vi "Dresden R2R Sputter 03.02.2018 IY24.vi"() -> ()   [LabVIEW 2009] (continued)
                                frame #1 {
                                n20568 = local read "Semi"() -> (w23364:bool)
                                n20569 = case shown="False" w23364 {
                                frame #0 {
                                n20570 = Wait (ms)(milliseconds to wait=u32 1000) -> ()  [unwired: 1 out]
                                n20571 = local write "Ch3_Sd3"(TRUE ("Ch1_Sd1 2")) -> ()
                                }
                                frame #1 {
                                }
                                }
                                }
                                }
                                }
                                frame #1 {
                                }
                                }
                              }
                              frame #4 {
                                n20572 = local read "Yes 3"() -> (w23367:bool)
                                n20573 = case shown="False" w23367 {
                                frame #0 {
                                # "CLOSE PC-BV"
                                n20574 = local read "Semi"() -> (w23368:bool)
                                n20575 = case shown="False" w23368 {
                                frame #0 {
                                n20576 = stacked-sequence {
                                frame #0 {
                                n20577 = local read "Semi"() -> (w23369:bool)
                                n20578 = case shown="False" w23369 {
                                frame #0 {
                                n20579 = stacked-sequence {
                                frame #0 {
                                n20580 = local read "Semi"() -> (w23370:bool)
                                n20581 = case shown="False" w23370 {
                                frame #0 {
                                n20582 = local write "Pc_bv3_auto_close"(TRUE ("Tp1_auto_start")) -> ()
                                }
                                frame #1 {
                                }
                                }
                                }
                                frame #1 {
                                n20583 = local read "Semi"() -> (w23372:bool)
                                n20584 = case shown="False" w23372 {
                                frame #0 {
                                n20585 = Wait (ms)(milliseconds to wait=u32 1000) -> ()  [unwired: 1 out]
                                }
                                frame #1 {
                                }
                                }
                                }
                                frame #2 {
                                n20586 = local read "Semi"() -> (w23374:bool)
                                n20587 = case shown="False" w23374 {
                                frame #0 {
                                n20588 = while {
                                i -> [w23380]
                                stop <- w23376 stop-if-true
                                n20589 = local read "Pc_bv_closed_ch3"() -> (w23378:bool)
                                n20590 = Greater?(x=w23380, y=120) -> (0:w23379:bool)
                                n20591 = local read "Semi"() -> (w23377:bool)
                                n20592 = Compound Arithmetic op=OR(w23377, w23378, w23379) -> (w23376:bool)
                                n20593 = Wait (ms)(milliseconds to wait=u32 500) -> ()  [unwired: 1 out]
                                }
                                }
                                frame #1 {
                                }
                                }
                                }
                                frame #3 {
                                n20594 = local read "Semi"() -> (w23382:bool)
                                n20595 = case shown="False" w23382 {
                                frame #0 {
                                n20596 = local read "Pc_bv_closed_ch3"() -> (w23383:bool)
                                n20597 = case shown="False" w23383 {
                                frame #0 {
                                n20598 = local write "Pc_bv3_auto_close"(TRUE ("Pc_bv1_auto_open")) -> ()
                                }
                                frame #1 {
                                }
                                }
                                }
                                frame #1 {
                                }
                                }
                                }
                                frame #4 {
                                n20599 = local read "Semi"() -> (w23385:bool)
                                n20600 = case shown="False" w23385 {
                                frame #0 {
                                n20601 = local read "Pc_bv_closed_ch3"() -> (w23386:bool)
                                n20602 = case shown="False" w23386 {
                                frame #0 {
                                n20603 = Wait (ms)(milliseconds to wait=u32 1000) -> ()  [unwired: 1 out]
                                }
                                frame #1 {
                                }
                                }
                                }
                                frame #1 {
                                }
                                }
                                }
                                frame #5 {
                                n20604 = local read "Semi"() -> (w23388:bool)
                                n20605 = case shown="False" w23388 {
                                frame #0 {
                                n20606 = while {
                                i -> [w23394]
                                stop <- w23390 stop-if-true
                                n20607 = local read "Pc_bv_closed_ch3"() -> (w23392:bool)
                                n20608 = Greater?(x=w23394, y=120) -> (0:w23393:bool)
                                n20609 = local read "Semi"() -> (w23391:bool)
                                n20610 = Compound Arithmetic op=OR(w23391, w23392, w23393) -> (w23390:bool)
                                n20611 = Wait (ms)(milliseconds to wait=u32 500) -> ()  [unwired: 1 out]
                                }
                                }
                                frame #1 {
                                }
                                }
                                }
                                frame #6 {
                                n20612 = local read "Semi"() -> (w23396:bool)
                                n20613 = case shown="False" w23396 {
                                frame #0 {
                                n20614 = local read "Pc_bv_closed_ch3"() -> (w23397:bool)
                                n20615 = case shown="False" w23397 {
                                frame #0 {
                                n20616 = local write "Error Message"("Shut Down process  cancelled\nbecause  PC-BV not opened.\nPlease check PC-BV3 connections." ("Error Message")) -> ()
                                n20617 = local write "Semi"(TRUE ("Semi")) -> ()
                                }
                                frame #1 {
                                }
                                }
                                }
                                frame #1 {
                                }
                                }
                                }
                                }
                                }
                                frame #1 {
                                }
                                }
                                }
                                frame #1 {
                                n20618 = local read "Semi"() -> (w23400:bool)
                                n20619 = case shown="False" w23400 {
                                frame #0 {
                                n20620 = local write "Ch3_Sd4"(TRUE ("Ch1_Sd2")) -> ()
                                n20621 = Wait (ms)(milliseconds to wait=u32 1000) -> ()  [unwired: 1 out]
                                }
                                frame #1 {
                                }
                                }
                                }
                                }
                                }
                                frame #1 {
                                }
                                }
                                }
                                frame #1 {
                                # "OPEN PC-BV"
                                n20622 = local read "Semi"() -> (w23403:bool)
                                n20623 = case shown="False" w23403 {
                                frame #0 {
                                n20624 = stacked-sequence {
                                frame #0 {
                                n20625 = local read "Semi"() -> (w23404:bool)
                                n20626 = case shown="False" w23404 {
                                frame #0 {
                                n20627 = stacked-sequence {
                                frame #0 {
                                n20628 = local read "Semi"() -> (w23405:bool)
                                n20629 = case shown="False" w23405 {
                                frame #0 {
                                n20630 = local write "Pc_bv3_auto_open"(TRUE ("Tp1_auto_start")) -> ()
                                }
                                frame #1 {
                                }
                                }
                                }
                                frame #1 {
                                n20631 = local read "Semi"() -> (w23407:bool)
                                n20632 = case shown="False" w23407 {
                                frame #0 {
                                n20633 = Wait (ms)(milliseconds to wait=u32 1000) -> ()  [unwired: 1 out]
                                }
                                frame #1 {
                                }
                                }
                                }
                                frame #2 {
                                n20634 = local read "Semi"() -> (w23409:bool)
                                n20635 = case shown="False" w23409 {
                                frame #0 {
                                n20636 = while {
                                i -> [w23415]
                                stop <- w23411 stop-if-true
                                n20637 = local read "Pc_bv_opened_ch3"() -> (w23413:bool)
                                n20638 = Greater?(x=w23415, y=120) -> (0:w23414:bool)
                                n20639 = local read "Semi"() -> (w23412:bool)
                                n20640 = Compound Arithmetic op=OR(w23412, w23413, w23414) -> (w23411:bool)
                                n20641 = Wait (ms)(milliseconds to wait=u32 500) -> ()  [unwired: 1 out]
                                }
                                }
                                frame #1 {
                                }
                                }
                                }
                                frame #3 {
                                n20642 = local read "Semi"() -> (w23417:bool)
                                n20643 = case shown="False" w23417 {
                                frame #0 {
                                n20644 = local read "Pc_bv_opened_ch3"() -> (w23418:bool)
                                n20645 = case shown="False" w23418 {
                                frame #0 {
                                n20646 = local write "Pc_bv3_auto_open"(TRUE ("Pc_bv1_auto_open")) -> ()
                                }
                                frame #1 {
                                }
                                }
                                }
                                frame #1 {
                                }
                                }
                                }
                                frame #4 {
                                n20647 = local read "Semi"() -> (w23420:bool)
                                n20648 = case shown="False" w23420 {
                                frame #0 {
                                n20649 = local read "Pc_bv_opened_ch3"() -> (w23421:bool)
                                n20650 = case shown="False" w23421 {
                                frame #0 {
                                n20651 = Wait (ms)(milliseconds to wait=u32 1000) -> ()  [unwired: 1 out]
                                }
                                frame #1 {
                                }
                                }
                                }
                                frame #1 {
                                }
                                }
                                }
                                frame #5 {
                                n20652 = local read "Semi"() -> (w23423:bool)
                                n20653 = case shown="False" w23423 {
                                frame #0 {
                                n20654 = while {
                                i -> [w23429]
                                stop <- w23425 stop-if-true
                                n20655 = local read "Pc_bv_opened_ch3"() -> (w23427:bool)
                                n20656 = Greater?(x=w23429, y=120) -> (0:w23428:bool)
                                n20657 = local read "Semi"() -> (w23426:bool)
                                n20658 = Compound Arithmetic op=OR(w23426, w23427, w23428) -> (w23425:bool)
                                n20659 = Wait (ms)(milliseconds to wait=u32 500) -> ()  [unwired: 1 out]
                                }
                                }
                                frame #1 {
                                }
                                }
                                }
                                frame #6 {
                                n20660 = local read "Semi"() -> (w23431:bool)
                                n20661 = case shown="False" w23431 {
                                frame #0 {
                                n20662 = local read "Pc_bv_opened_ch3"() -> (w23432:bool)
                                n20663 = case shown="False" w23432 {
                                frame #0 {
                                n20664 = local write "Error Message"("Shut Down process  cancelled\nbecause  PC-BV not opened.\nPlease check PC-BV3 connections." ("Error Message")) -> ()
                                n20665 = Wait (ms)(milliseconds to wait=u32 1000) -> ()  [unwired: 1 out]
                                }
                                frame #1 {
                                }
                                }
                                }
                                frame #1 {
                                }
                                }
                                }
                                }
                                }
                                frame #1 {
                                }
                                }
                                }
                                frame #1 {
                                n20666 = local read "Semi"() -> (w23435:bool)
                                n20667 = case shown="False" w23435 {
                                frame #0 {
                                n20668 = local write "Ch3_Sd5"(TRUE ("Ch1_Sd2")) -> ()
                                n20669 = Wait (ms)(milliseconds to wait=u32 1000) -> ()  [unwired: 1 out]
                                }
                                frame #1 {
                                }
                                }
                                }
                                }
                                }
                                frame #1 {
                                }
                                }
                                }
                                }
                              }
                              frame #5 {
                                # "CLOSE TP-BV"
                                n20670 = local read "Semi"() -> (w23438:bool)
                                n20671 = case shown="False" w23438 {
                                frame #0 {
                                n20672 = stacked-sequence {
                                frame #0 {
                                n20673 = local read "Semi"() -> (w23439:bool)
                                n20674 = case shown="False" w23439 {
                                frame #0 {
                                n20675 = while {
                                i -> [w23445]
                                stop <- w23440 stop-if-true
                                n20676 = Greater?(x=w23445, y=25) -> (0:w23444:bool)
                                n20677 = case shown="True" w23444 {
                                frame #0 {
                                }
                                frame #1 {
                                n20678 = local write "Error Message"("Shut Down Process  cancelled\nbecause  TP-BV not closed.\nPlease check TP-BV3  connections." ("Error Message")) -> ()
                                n20679 = local write "Semi"(TRUE ("Semi")) -> ()
                                }
                                }
                                n20680 = local read "Ch3_Tp_bv_di"() -> (w23443:bool)
                                n20681 = case shown="True" w23443 {
                                tunnel: [TRUE FALSE] -> w23441
                                frame #0 {
                                }
                                frame #1 {
                                n20682 = Wait Until Next ms Multiple(millisecond multiple=u32 200) -> ()  [unwired: 1 out]
                                n20683 = local write "Ch3_Tp_bv_do"(FALSE ("Ch1_Ch_cc_on_off_di")) -> ()
                                }
                                }
                                n20684 = local read "Semi"() -> (w23442:bool)
                                n20685 = Or(x=w23441, y=w23442) -> (x .or. y?=w23440:bool)
                                }
                                }
                                frame #1 {
                                }
                                }
                                }
                                frame #1 {
                                n20686 = local read "Semi"() -> (w23453:bool)
                                n20687 = case shown="False" w23453 {
                                frame #0 {
                                n20688 = local write "Ch3_Sd6"(TRUE ("Ch1_Sd5")) -> ()
                                n20689 = Wait (ms)(milliseconds to wait=u32 1000) -> ()  [unwired: 1 out]
                                }
                                frame #1 {
                                }
                                }
                                }
                                }
                                }
                                frame #1 {
                                }
                                }
                              }
                              frame #6 {
                                # "STOP MP"
                                n20690 = local read "Semi"() -> (w23456:bool)
                                n20691 = case shown="False" w23456 {
                                frame #0 {
                                n20692 = stacked-sequence {
                                frame #0 {
                                n20693 = local read "Semi"() -> (w23457:bool)
                                n20694 = case shown="False" w23457 {
                                frame #0 {
                                n20695 = while {
                                i -> [w23463]
                                stop <- w23458 stop-if-true
                                n20696 = Greater?(x=w23463, y=25) -> (0:w23462:bool)
                                n20697 = case shown="True" w23462 {
                                frame #0 {
                                }
                                frame #1 {
                                n20698 = local write "Error Message"("Shut Down Process  cancelled\nbecause  MP not closed.\nPlease check MP3 connections." ("Error Message")) -> ()
                                n20699 = local write "Semi"(TRUE ("Semi")) -> ()
                                }
                                }
                                n20700 = local read "Ch3_Mp_di"() -> (w23461:bool)
                                n20701 = case shown="True" w23461 {
                                tunnel: [TRUE FALSE] -> w23459
                                frame #0 {
                                }
                                frame #1 {
                                n20702 = Wait Until Next ms Multiple(millisecond multiple=u32 200) -> ()  [unwired: 1 out]
                                n20703 = local write "Ch3_Mp_do"(FALSE ("Ch1_Ch_cc_on_off_di")) -> ()
                                }
                                }
                                n20704 = local read "Semi"() -> (w23460:bool)
                                n20705 = Or(x=w23459, y=w23460) -> (x .or. y?=w23458:bool)
                                }
                                }
                                frame #1 {
                                }
                                }
                                }
                                frame #1 {
                                n20706 = local read "Semi"() -> (w23471:bool)
                                n20707 = case shown="False" w23471 {
                                frame #0 {
                                n20708 = local write "Ch3_Sd7"(TRUE ("Ch1_Sd6")) -> ()
                                n20709 = Wait (ms)(milliseconds to wait=u32 1000) -> ()  [unwired: 1 out]
                                }
                                frame #1 {
                                }
                                }
                                }
                                }
                                }
                                frame #1 {
                                }
                                }
                              }
                              frame #7 {
                                # "PL-VBV OPEN  & CHECK"
                                n20710 = local read "Semi"() -> (w23474:bool)
                                n20711 = case shown="False" w23474 {
                                frame #0 {
                                n20712 = stacked-sequence {
                                frame #0 {
                                n20713 = local read "Semi"() -> (w23475:bool)
                                n20714 = case shown="False" w23475 {
                                frame #0 {
                                n20715 = local write "Ch3_Pl_atm_do"(FALSE ("Ch1_Pl_atm_do")) -> ()
                                n20716 = Wait Until Next ms Multiple(millisecond multiple=u32 2000) -> ()  [unwired: 1 out]
                                }
                                frame #1 {
                                }
                                }
                                }
                                frame #1 {
                                n20717 = local read "Semi"() -> (w23478:bool)
                                n20718 = case shown="False" w23478 {
                                frame #0 {
                                n20719 = while {
                                i -> [w23484]
                                stop <- w23480 stop-if-true
                                n20720 = Greater?(x=w23484, y=50) -> (0:w23483:bool)
                                n20721 = case shown="True" w23483 {
                                frame #0 {
                                }
                                frame #1 {
                                n20722 = local write "Error Message"("Shut Down Process  cancelled\nbecause  PL-VBV not opened.\nPlease check  PL-VBV3 connections." ("Error Message")) -> ()
                                n20723 = local write "Semi"(TRUE ("Semi")) -> ()
                                }
                                }
                                n20724 = local read "Ch3_Pl_atm_di"() -> (w23479:bool)
                                n20725 = case shown="False" w23479 {
                                tunnel: [w23486 TRUE] -> w23481
                                frame #0 {
                                n20726 = local read "Ch3_Pl_vbv_di"() -> (w23487:bool)
                                n20727 = case shown="False" w23487 {
                                tunnel: [FALSE TRUE] -> w23486
                                frame #0 {
                                n20728 = Wait Until Next ms Multiple(millisecond multiple=u32 500) -> ()  [unwired: 1 out]
                                n20729 = local write "Ch3_Pl_vbv_do"(TRUE ("Ch1_Ch_cc_on_off_di")) -> ()
                                }
                                frame #1 {
                                }
                                }
                                }
                                frame #1 {
                                n20730 = Wait Until Next ms Multiple(millisecond multiple=u32 500) -> ()  [unwired: 1 out]
                                }
                                }
                                n20731 = local read "Semi"() -> (w23482:bool)
                                n20732 = Or(x=w23481, y=w23482) -> (x .or. y?=w23480:bool)
                                }
                                }
                                frame #1 {
                                }
                                }
                                }
                                frame #2 {
                                n20733 = local read "Semi"() -> (w23496:bool)
                                n20734 = case shown="False" w23496 {
                                frame #0 {
                                n20735 = local write "Ch3_Sd8"(TRUE ("Ch1_Sd8")) -> ()
                                n20736 = Wait (ms)(milliseconds to wait=u32 1000) -> ()  [unwired: 1 out]
                                }
                                frame #1 {
                                }
                                }
                                }
                                }
                                }
                                frame #1 {
                                }
                                }
                              }
                              frame #8 {
                                # "PL-VBV CLOSE  & CHECK"
                                n20737 = local read "Semi"() -> (w23499:bool)
                                n20738 = case shown="False" w23499 {
                                frame #0 {
                                n20739 = stacked-sequence {
                                frame #0 {
                                n20740 = local read "Semi"() -> (w23500:bool)
                                n20741 = case shown="False" w23500 {
                                frame #0 {
                                n20742 = while {
                                i -> [w23506]
                                stop <- w23502 stop-if-true
                                n20743 = Greater?(x=w23506, y=50) -> (0:w23505:bool)
                                n20744 = case shown="True" w23505 {
                                frame #0 {
                                }
                                frame #1 {
                                n20745 = local write "Error Message"("Shut Down Process  cancelled\nbecause  PL-VBV not closed.\nPlease check PL-VBV3 connections." ("Error Message")) -> ()
                                n20746 = local write "Semi"(TRUE ("Semi")) -> ()
                                }
                                }
                                n20747 = local read "Ch3_Pl_atm_di"() -> (w23501:bool)
                                n20748 = case shown="True" w23501 {
                                tunnel: [FALSE w23510] -> w23503
                                frame #0 {
                                n20749 = Wait Until Next ms Multiple(millisecond multiple=u32 500) -> ()  [unwired: 1 out]
                                }
                                frame #1 {
                                n20750 = local read "Ch3_Pl_vbv_di"() -> (w23511:bool)
                                n20751 = case shown="True" w23511 {
                                tunnel: [TRUE FALSE] -> w23510
                                frame #0 {
                                }
                                frame #1 {
                                n20752 = Wait Until Next ms Multiple(millisecond multiple=u32 500) -> ()  [unwired: 1 out]
                                n20753 = local write "Ch3_Pl_vbv_do"(FALSE ("Ch1_Ch_cc_on_off_di")) -> ()
                                }
                                }
                                }
                                }
                                n20754 = local read "Semi"() -> (w23504:bool)
                                n20755 = Or(x=w23503, y=w23504) -> (x .or. y?=w23502:bool)
                                }
                                }
                                frame #1 {
                                }
                                }
                                }
                                frame #1 {
                                n20756 = local read "Semi"() -> (w23518:bool)
                                n20757 = case shown="False" w23518 {
                                frame #0 {
                                n20758 = local write "Ch3_Sd9"(TRUE ("Ch1_Sd11")) -> ()
                                n20759 = Wait (ms)(milliseconds to wait=u32 1000) -> ()  [unwired: 1 out]
                                }
                                frame #1 {
                                }
                                }
                                }
                                }
                                }
                                frame #1 {
                                }
                                }
                              }
                              frame #9 {
                                # "WAIT DECELARATING TP"
                                n20760 = local read "Semi"() -> (w23521:bool)
                                n20761 = case shown="False" w23521 {
                                frame #0 {
                                n20762 = stacked-sequence {
                                frame #0 {
                                n20763 = local read "Semi"() -> (w23522:bool)
                                n20764 = case shown="False" w23522 {
                                frame #0 {
                                n20765 = while {
                                i -> [w23528]
                                stop <- w23524 stop-if-true
                                n20766 = Greater?(x=w23528, y=1500) -> (0:w23527:bool)
                                n20767 = case shown="True" w23527 {
                                frame #0 {
                                }
                                frame #1 {
                                n20768 = local write "Error Message"("Shut Down Process  cancelled\nbecause TP not decelarating.\nPlease check TP3 connections." ("Error Message")) -> ()
                                n20769 = local write "Semi"(TRUE ("Semi")) -> ()
                                }
                                }
                                n20770 = local read "Yes 3"() -> (w23523:bool)
                                n20771 = case shown="True" w23523 {
                                tunnel: [TRUE w23534] -> w23525
                                frame #0 {
                                }
                                frame #1 {
                                n20772 = local read "Tp3_speed_gui"() -> (w23532:i32)
                                n20773 = Less?(x=w23532, y="Tp3_safety_speed") -> (x < y?=w23531:bool)
                                n20774 = case shown="False" w23531 {
                                tunnel: [FALSE TRUE] -> w23534
                                frame #0 {
                                n20775 = Wait Until Next ms Multiple(millisecond multiple=u32 500) -> ()  [unwired: 1 out]
                                }
                                frame #1 {
                                }
                                }
                                }
                                }
                                n20776 = local read "Semi"() -> (w23526:bool)
                                n20777 = Or(x=w23525, y=w23526) -> (x .or. y?=w23524:bool)
                                }
                                }
                                frame #1 {
                                }
                                }
                                }
                                frame #1 {
                                n20778 = local read "Semi"() -> (w23540:bool)
                                n20779 = case shown="False" w23540 {
                                frame #0 {
                                n20780 = Wait (ms)(milliseconds to wait=u32 1000) -> ()  [unwired: 1 out]
                                n20781 = local write "Ch3_Sd10"(TRUE ("Ch1_Sd3")) -> ()
                                }
                                frame #1 {
                                }
                                }
                                }
                                }
                                }
                                frame #1 {
                                }
                                }
                              }
                              frame #10 {
                                # "CH-VBV OPEN  & CHECK"
                                n20782 = local read "Yes 3"() -> (w23543:bool)
                                n20783 = case shown="True" w23543 {
                                frame #0 {
                                }
                                frame #1 {
                                n20784 = local read "Semi"() -> (w23544:bool)
                                n20785 = case shown="False" w23544 {
                                frame #0 {
                                n20786 = stacked-sequence {
                                frame #0 {
                                n20787 = local read "Semi"() -> (w23545:bool)
                                n20788 = case shown="False" w23545 {
                                frame #0 {
                                n20789 = local write "Ch3_Ch_atm_do"(FALSE ("Ch1_Pl_atm_do")) -> ()
                                n20790 = Wait Until Next ms Multiple(millisecond multiple=u32 2000) -> ()  [unwired: 1 out]
                                }
                                frame #1 {
                                }
                                }
                                }
                                frame #1 {
                                n20791 = local read "Semi"() -> (w23548:bool)
                                n20792 = case shown="False" w23548 {
                                frame #0 {
                                n20793 = while {
                                i -> [w23554]
                                stop <- w23550 stop-if-true
                                n20794 = Greater?(x=w23554, y=50) -> (0:w23553:bool)
                                n20795 = case shown="True" w23553 {
                                frame #0 {
                                }
                                frame #1 {
                                n20796 = local write "Error Message"("Shut Down Process  cancelled\nbecause  CH-VBV not opened.\nPlease check  CH-VBV3  connections." ("Error Message")) -> ()
                                n20797 = local write "Semi"(TRUE ("Semi")) -> ()
                                }
                                }
                                n20798 = local read "Ch3_Ch_atm_di"() -> (w23549:bool)
                                n20799 = case shown="False" w23549 {
                                tunnel: [w23556 TRUE] -> w23551
                                frame #0 {
                                n20800 = local read "Ch3_Ch_vbv_di"() -> (w23557:bool)
                                n20801 = case shown="False" w23557 {
                                tunnel: [FALSE TRUE] -> w23556
                                frame #0 {
                                n20802 = Wait Until Next ms Multiple(millisecond multiple=u32 200) -> ()  [unwired: 1 out]
                                n20803 = local write "Ch3_Ch_vbv_do"(TRUE ("Ch1_Ch_cc_on_off_di")) -> ()
                                }
                                frame #1 {
                                }
                                }
                                }
                                frame #1 {
                                }
                                }
                                n20804 = local read "Semi"() -> (w23552:bool)
                                n20805 = Or(x=w23551, y=w23552) -> (x .or. y?=w23550:bool)
                                }
                                }
                                frame #1 {
                                }
                                }
                                }
                                frame #2 {
                                n20806 = local read "Semi"() -> (w23565:bool)
                                n20807 = case shown="False" w23565 {
                                frame #0 {
                                n20808 = Wait (ms)(milliseconds to wait=u32 1000) -> ()  [unwired: 1 out]
                                n20809 = local write "Ch3_Sd11"(TRUE ("Ch1_Sd9")) -> ()
                                }
                                frame #1 {
                                }
                                }
                                }
                                }
                                }
                                frame #1 {
                                }
                                }
                                }
                                }
                              }
                              frame #11 {
                                # "CH-VBV CLOSE &  CHECK"
                                n20810 = local read "Yes 3"() -> (w23568:bool)
                                n20811 = case shown="True" w23568 {
                                frame #0 {
                                }
                                frame #1 {
                                n20812 = local read "Semi"() -> (w23569:bool)
                                n20813 = case shown="False" w23569 {
                                frame #0 {
                                n20814 = stacked-sequence {
                                frame #0 {
                                n20815 = local read "Semi"() -> (w23570:bool)
                                n20816 = case shown="False" w23570 {
                                frame #0 {
                                n20817 = while {
                                i -> [w23578]
                                stop <- w23574 stop-if-true
                                n20818 = Greater?(x=w23578, y=50) -> (0:w23577:bool)
                                n20819 = case shown="True" w23577 {
                                frame #0 {
                                }
                                frame #1 {
                                n20820 = local write "Error Message"("Shut Down Process  cancelled\nbecause  CH-VBV  not closed.\nPlease check CH-VBV3 connections." ("Error Message")) -> ()
                                n20821 = local write "Semi"(TRUE ("Semi")) -> ()
                                }
                                }
                                n20822 = local read "Tp3_speed_gui"() -> (w23572:i32)
                                n20823 = Greater Or Equal?(x=w23572, y=u64 100) -> (x >= y?=w23571:bool)
                                n20824 = case shown="True" w23571 {
                                tunnel: [TRUE w23581] -> w23575
                                frame #0 {
                                }
                                frame #1 {
                                n20825 = local read "Ch3_Ch_vbv_di"() -> (w23582:bool)
                                n20826 = case shown="True" w23582 {
                                tunnel: [TRUE FALSE] -> w23581
                                frame #0 {
                                }
                                frame #1 {
                                n20827 = Wait Until Next ms Multiple(millisecond multiple=u32 500) -> ()  [unwired: 1 out]
                                n20828 = local write "Ch3_Ch_vbv_do"(FALSE ("Ch1_Ch_cc_on_off_di")) -> ()
                                }
                                }
                                }
                                }
                                n20829 = local read "Semi"() -> (w23576:bool)
                                n20830 = Or(x=w23575, y=w23576) -> (x .or. y?=w23574:bool)
                                }
                                }
                                frame #1 {
                                }
                                }
                                }
                                frame #1 {
                                n20831 = local read "Semi"() -> (w23589:bool)
                                n20832 = case shown="False" w23589 {
                                frame #0 {
                                n20833 = local write "Ch3_Sd12"(TRUE ("Ch1_Sd13")) -> ()
                                n20834 = Wait (ms)(milliseconds to wait=u32 1000) -> ()  [unwired: 1 out]
                                }
                                frame #1 {
                                }
                                }
                                }
                                frame #2 {
                                n20835 = local read "Semi"() -> (w23592:bool)
                                n20836 = case shown="False" w23592 {
                                frame #0 {
                                n20837 = Wait (ms)(milliseconds to wait=u32 3000) -> ()  [unwired: 1 out]
                                }
                                frame #1 {
                                }
                                }
                                }
                                }
                                }
                                frame #1 {
                                }
                                }
                                }
                                }
                              }
                              frame #12 {
                                # "CH-VBV OPEN &  CHECK"
                                n20838 = local read "Yes 3"() -> (w23594:bool)
                                n20839 = case shown="True" w23594 {
                                frame #0 {
                                }
                                frame #1 {
                                n20840 = local read "Semi"() -> (w23595:bool)
                                n20841 = case shown="False" w23595 {
                                frame #0 {
                                n20842 = stacked-sequence {
                                frame #0 {
                                n20843 = local read "Semi"() -> (w23596:bool)
                                n20844 = case shown="False" w23596 {
                                frame #0 {
                                n20845 = while {
                                i -> [w23602]
                                stop <- w23598 stop-if-true
                                n20846 = Greater?(x=w23602, y=200) -> (0:w23601:bool)
                                n20847 = case shown="True" w23601 {
                                frame #0 {
                                }
                                frame #1 {
                                n20848 = local write "Error Message"("Shut Down Process  cancelled\nbecause  CH-VBV  not opened.\nPlease check CH-VBV3 connections." ("Error Message")) -> ()
                                n20849 = local write "Semi"(TRUE ("Semi")) -> ()
                                }
                                }
                                n20850 = local read "Ch3_Ch_vbv_di"() -> (w23597:bool)
                                n20851 = case shown="False" w23597 {